vi "FlexMag - 23-03-2023.vi"() -> ()   [LabVIEW 2018] (continued)
                                stop <- w20767 stop-if-true
                                n15578 = Greater Or Equal?(x=w20771, y=200) -> (x >= y?=w20773:bool)
                                n15579 = case shown="True" w20773 {
                                frame False {
                                }
                                frame True {
                                n15580 = local write "ch2 pumpdown error"(TRUE ("ch1 pumpdown error")) -> ()
                                n15581 = local write "Warning Message"("CH2 PumpDown process  is canceled !\nCH2 PC GV couldn't be opened" ("Warning Message")) -> ()
                                }
                                }
                                n15582 = local read "ch2 pumpdown alg"() -> (w20770:bool)
                                n15583 = local read "ch2_pcgv_gui"() -> (w20766:bool)
                                n15584 = local read "abort ch2"() -> (w20768:bool)
                                n15585 = Wait Until Next ms Multiple(millisecond multiple=u32 200) -> ()  [unwired: 1 out]
                                n15586 = Not(x=w20770) -> (.not. x?=w20769:bool)
                                n15587 = Compound Arithmetic op=OR(w20766, w20768, w20769) -> (w20767:bool)
                                }
                                }
                                }
                              }
                              frame #4 {
                                n15588 = local read "ch2 pumpdown alg"() -> (w20776:bool)
                                n15589 = case shown="True" w20776 {
                                frame False {
                                }
                                frame True {
                                n15590 = local write "ch2 pc gv open led"(TRUE ("ch1 tp bv open led")) -> ()
                                n15591 = Wait (ms)(milliseconds to wait=u32 1000) -> ()  [unwired: 1 out]
                                }
                                }
                              }
                            }
                          }
                        }
                      }
                      frame True {
                      }
                    }
                  }
                }
              }
              frame #16 {
                n15592 = stacked-sequence {
                  frame #0 {
                    n15593 = local read "ch2 pumpdown alg"() -> (w20779:bool)
                    n15594 = case shown="True" w20779 {
                      frame False {
                      }
                      frame True {
                        n15595 = local read "abort ch2"() -> (w20780:bool)
                        n15596 = case shown="False" w20780 {
                          frame False {
                            n15597 = local write "CH2_PL_ATM_DO"(TRUE ("CH1_PL_ATM_DO")) -> ()
                            n15598 = Wait (ms)(milliseconds to wait=u32 2000) -> ()  [unwired: 1 out]
                          }
                          frame True {
                          }
                        }
                      }
                    }
                  }
                  frame #1 {
                    n15599 = local read "ch2 pumpdown alg"() -> (w20783:bool)
                    n15600 = case shown="True" w20783 {
                      frame False {
                      }
                      frame True {
                        n15601 = local read "abort ch2"() -> (w20784:bool)
                        n15602 = case shown="False" w20784 {
                          frame False {
                            n15603 = local write "CH2_CH_ATM_DO"(TRUE ("CH1_CH_ATM_DO")) -> ()
                            n15604 = Wait (ms)(milliseconds to wait=u32 2000) -> ()  [unwired: 1 out]
                          }
                          frame True {
                          }
                        }
                      }
                    }
                  }
                }
              }
              frame #17 {
                # "mp start"
                n15605 = local read "ch2 pumpdown alg"() -> (w20787:bool)
                n15606 = case shown="True" w20787 {
                  frame False {
                  }
                  frame True {
                    n15607 = local read "abort ch2"() -> (w20788:bool)
                    n15608 = case shown="False" w20788 {
                      frame False {
                        n15609 = while {
                          i -> [w20793]
                          stop <- w20797 stop-if-true
                          n15610 = Greater?(x=w20793, y=100) -> (0:w20789:bool)
                          n15611 = case shown="True" w20789 {
                            frame False {
                            }
                            frame True {
                              n15612 = local write "Warning Message"("CH2 PumpDown process  is canceled !\nCH2 MP couldn't be started" ("Warning Message")) -> ()
                              n15613 = local write "ch2 pumpdown error"(TRUE ("ch1 pumpdown error")) -> ()
                            }
                          }
                          n15614 = local read "CH2_MP_DI"() -> (w20791:bool)
                          n15615 = case shown="False" w20791 {
                            tunnel: [FALSE TRUE] -> w20790
                            frame False {
                              n15616 = Wait Until Next ms Multiple(millisecond multiple=u32 200) -> ()  [unwired: 1 out]
                              n15617 = local write "CH2_MP_DO"(TRUE ("CH1_MP_DO")) -> ()
                            }
                            frame True {
                            }
                          }
                          n15618 = local read "ch2 pumpdown alg"() -> (w20796:bool)
                          n15619 = local read "abort ch2"() -> (w20794:bool)
                          n15620 = Not(x=w20796) -> (.not. x?=w20795:bool)
                          n15621 = Compound Arithmetic op=OR(w20790, w20794, w20795) -> (w20797:bool)
                        }
                      }
                      frame True {
                      }
                    }
                  }
                }
              }
              frame #18 {
                n15622 = local read "ch2 pumpdown alg"() -> (w20804:bool)
                n15623 = case shown="True" w20804 {
                  frame False {
                  }
                  frame True {
                    n15624 = local read "abort ch2"() -> (w20805:bool)
                    n15625 = case shown="False" w20805 {
                      frame False {
                        n15626 = local write "ch2 mp start led"(TRUE ("ch1 ch vbv close")) -> ()
                        n15627 = Wait (ms)(milliseconds to wait=u32 1000) -> ()  [unwired: 1 out]
                      }
                      frame True {
                      }
                    }
                  }
                }
              }
              frame #19 {
                # "pl pg check"
                n15628 = local read "ch2 pumpdown alg"() -> (w20808:bool)
                n15629 = case shown="True" w20808 {
                  frame False {
                  }
                  frame True {
                    n15630 = local read "abort ch2"() -> (w20809:bool)
                    n15631 = case shown="False" w20809 {
                      frame False {
                        n15632 = while {
                          i -> [w20816]
                          stop <- w20820 stop-if-true
                          # "30 min"
                          n15633 = Greater?(x=w20816, y=9000) -> (0:w20813:bool)
                          n15634 = case shown="True" w20813 {
                            frame False {
                            }
                            frame True {
                              n15635 = local write "Warning Message"("CH2 PumpDown process  is canceled !\nCH2 PL Pressure couldn't be reached under 0.5 Torr" ("Warning Message")) -> ()
                              n15636 = local write "ch2 pumpdown error"(TRUE ("ch1 pumpdown error")) -> ()
                            }
                          }
                          n15637 = local read "ch2 pl pg  torr"() -> (w20812:dbl)
                          n15638 = Less?(x=w20812, y=0.7) -> (x < y?=w20810:bool)
                          n15639 = case shown="False" w20810 {
                            tunnel: [FALSE TRUE] -> w20814
                            frame False {
                              n15640 = Wait Until Next ms Multiple(millisecond multiple=u32 200) -> ()  [unwired: 1 out]
                            }
                            frame True {
                            }
                          }
                          n15641 = local read "ch2 pumpdown alg"() -> (w20819:bool)
                          n15642 = local read "abort ch2"() -> (w20817:bool)
                          n15643 = Not(x=w20819) -> (.not. x?=w20818:bool)
                          n15644 = Compound Arithmetic op=OR(w20814, w20817, w20818) -> (w20820:bool)
                        }
                      }
                      frame True {
                      }
                    }
                  }
                }
              }
              frame #20 {
                n15645 = local read "ch2 pumpdown alg"() -> (w20826:bool)
                n15646 = case shown="True" w20826 {
                  frame False {
                  }
                  frame True {
                    n15647 = local read "abort ch2"() -> (w20827:bool)
                    n15648 = case shown="False" w20827 {
                      frame False {
                        n15649 = local write "ch2 pl press under 0.05 T led"(TRUE ("ch1 ch vbv close")) -> ()
                        n15650 = Wait (ms)(milliseconds to wait=u32 1000) -> ()  [unwired: 1 out]
                      }
                      frame True {
                      }
                    }
                  }
                }
              }
              frame #21 {
                # "tp bv open"
                n15651 = local read "ch2 pumpdown alg"() -> (w20830:bool)
                n15652 = case shown="True" w20830 {
                  frame False {
                  }
                  frame True {
                    n15653 = local read "abort ch2"() -> (w20831:bool)
                    n15654 = case shown="False" w20831 {
                      frame False {
                        n15655 = while {
                          i -> [w20836]
                          stop <- w20840 stop-if-true
                          n15656 = Greater?(x=w20836, y=100) -> (0:w20832:bool)
                          n15657 = case shown="True" w20832 {
                            frame False {
                            }
                            frame True {
                              n15658 = local write "Warning Message"("CH2 PumpDown process  is canceled !\nCH2 TP BV couldn't be opened" ("Warning Message")) -> ()
                              n15659 = local write "ch2 pumpdown error"(TRUE ("ch1 pumpdown error")) -> ()
                            }
                          }
                          n15660 = local read "CH2_TP_BV_DI"() -> (w20834:bool)
                          n15661 = case shown="False" w20834 {
                            tunnel: [FALSE TRUE] -> w20833
                            frame False {
                              n15662 = Wait Until Next ms Multiple(millisecond multiple=u32 200) -> ()  [unwired: 1 out]
                              n15663 = local write "CH2_TP_BV_DO"(TRUE ("CH1_MP_DO")) -> ()
                            }
                            frame True {
                            }
                          }
                          n15664 = local read "ch2 pumpdown alg"() -> (w20839:bool)
                          n15665 = local read "abort ch2"() -> (w20837:bool)
                          n15666 = Not(x=w20839) -> (.not. x?=w20838:bool)
                          n15667 = Compound Arithmetic op=OR(w20833, w20837, w20838) -> (w20840:bool)
                        }
                      }
                      frame True {
                      }
                    }
                  }
                }
              }
              frame #22 {
                n15668 = local read "ch2 pumpdown alg"() -> (w20847:bool)
                n15669 = case shown="True" w20847 {
                  frame False {
                  }
                  frame True {
                    n15670 = local read "abort ch2"() -> (w20848:bool)
                    n15671 = case shown="False" w20848 {
                      frame False {
                        n15672 = local write "ch2 tp bv open led"(TRUE ("ch1 ch vbv close")) -> ()
                        n15673 = Wait (ms)(milliseconds to wait=u32 1000) -> ()  [unwired: 1 out]
                      }
                      frame True {
                      }
                    }
                  }
                }
              }
              frame #23 {
                # "pc gv open"
                n15674 = local read "ch2 pumpdown alg"() -> (w20851:bool)
                n15675 = case shown="True" w20851 {
                  frame False {
                  }
                  frame True {
                    n15676 = local read "abort ch2"() -> (w20852:bool)
                    n15677 = case shown="False" w20852 {
                      frame False {
                        n15678 = stacked-sequence {
                          frame #0 {
                            n15679 = local read "ch2 pumpdown alg"() -> (w20853:bool)
                            n15680 = case shown="True" w20853 {
                              frame False {
                              }
                              frame True {
                                n15681 = flat-sequence {
                                frame #0 {
                                n15682 = local write "pcgv2 auto open"(TRUE ("pcgv1 auto open")) -> ()
                                }
                                frame #1 {
                                n15683 = Wait (ms)(milliseconds to wait=u32 2000) -> ()  [unwired: 1 out]
                                }
                                frame #2 {
                                n15684 = local write "pcgv2 auto open"(TRUE ("pcgv1 auto open")) -> ()
                                }
                                }
                              }
                            }
                          }
                          frame #1 {
                            n15685 = while {
                              i -> [w20863]
                              stop <- w20859 stop-if-true
                              n15686 = Greater Or Equal?(x=w20863, y=200) -> (x >= y?=w20865:bool)
                              n15687 = case shown="True" w20865 {
                                frame False {
                                }
                                frame True {
                                n15688 = local write "ch2 pumpdown error"(TRUE ("ch1 pumpdown error")) -> ()
                                n15689 = local write "Warning Message"("CH2 PumpDown process  is canceled !\nCH2 PC GV couldn't be opened" ("Warning Message")) -> ()
                                }
                              }
                              n15690 = local read "ch2 pumpdown alg"() -> (w20862:bool)
                              n15691 = local read "ch2_pcgv_gui"() -> (w20858:bool)
                              n15692 = local read "abort ch2"() -> (w20860:bool)
                              n15693 = Wait Until Next ms Multiple(millisecond multiple=u32 200) -> ()  [unwired: 1 out]
                              n15694 = Not(x=w20862) -> (.not. x?=w20861:bool)
                              n15695 = Compound Arithmetic op=OR(w20858, w20860, w20861) -> (w20859:bool)
                            }
                          }
                        }
                      }
                      frame True {
                      }
                    }
                  }
                }
              }
              frame #24 {
                n15696 = local read "ch2 pumpdown alg"() -> (w20868:bool)
                n15697 = case shown="True" w20868 {
                  frame False {
                  }
                  frame True {
                    n15698 = local read "abort ch2"() -> (w20869:bool)
                    n15699 = case shown="False" w20869 {
                      frame False {
                        n15700 = local write "ch2 pc gv open led"(TRUE ("ch1 ch vbv close")) -> ()
                        n15701 = Wait (ms)(milliseconds to wait=u32 1000) -> ()  [unwired: 1 out]
                      }
                      frame True {
                      }
                    }
                  }
                }
              }
              frame #25 {
                # "ch pressure check"
                n15702 = local read "ch2 pumpdown alg"() -> (w20872:bool)
                n15703 = case shown="True" w20872 {
                  frame False {
                  }
                  frame True {
                    n15704 = local read "abort ch2"() -> (w20873:bool)
                    n15705 = case shown="False" w20873 {
                      frame False {
                        n15706 = while {
                          i -> [w20880]
                          stop <- w20884 stop-if-true
                          # "30 min"
                          n15707 = Greater?(x=w20880, y=9000) -> (0:w20877:bool)
                          n15708 = case shown="True" w20877 {
                            frame False {
                            }
                            frame True {
                              n15709 = local write "Warning Message"("CH2 PumpDown process  is canceled !\nCH2 CH Pressure couldn't be reached under 0.5 Torr" ("Warning Message")) -> ()
                              n15710 = local write "ch2 pumpdown error"(TRUE ("ch1 pumpdown error")) -> ()
                            }
                          }
                          n15711 = local read "ch2 ch pg torr"() -> (w20876:dbl)
                          n15712 = Less Or Equal?(x=w20876, y=0.5) -> (x <= y?=w20874:bool)
                          n15713 = case shown="False" w20874 {
                            tunnel: [FALSE TRUE] -> w20878
                            frame False {
                              n15714 = Wait Until Next ms Multiple(millisecond multiple=u32 200) -> ()  [unwired: 1 out]
                            }
                            frame True {
                            }
                          }
                          n15715 = local read "ch2 pumpdown alg"() -> (w20883:bool)
                          n15716 = local read "abort ch2"() -> (w20881:bool)
                          n15717 = Not(x=w20883) -> (.not. x?=w20882:bool)
                          n15718 = Compound Arithmetic op=OR(w20878, w20881, w20882) -> (w20884:bool)
                        }
                      }
                      frame True {
                      }
                    }
                  }
                }
              }
              frame #26 {
                n15719 = local read "ch2 pumpdown alg"() -> (w20890:bool)
                n15720 = case shown="True" w20890 {
                  frame False {
                  }
                  frame True {
                    n15721 = local read "abort ch2"() -> (w20891:bool)
                    n15722 = case shown="False" w20891 {
                      frame False {
                        n15723 = local write "ch2 ch press under 0.5 T led"(TRUE ("ch1 ch pressure led")) -> ()
                        n15724 = Wait (ms)(milliseconds to wait=u32 1000) -> ()  [unwired: 1 out]
                      }
                      frame True {
                      }
                    }
                  }
                }
              }
              frame #27 {
                # "ch 1 pressure check\nfor trns bp bv"
                n15725 = local read "ch2 pumpdown alg"() -> (w20894:bool)
                n15726 = case shown="True" w20894 {
                  frame False {
                  }
                  frame True {
                    n15727 = local read "abort ch2"() -> (w20895:bool)
                    n15728 = case shown="False" w20895 {
                      frame False {
                        n15729 = local read "ch1 ch pg torr"() -> (w20898:dbl)
                        n15730 = Less Or Equal?(x=w20898, y=0.5) -> (x <= y?=w20896:bool)
                        n15731 = case shown="True" w20896 {
                          frame False {
                          }
                          frame True {
                            n15732 = stacked-sequence {
                              frame #0 {
                                n15733 = while {
                                i -> [w20903]
                                stop <- w20907 stop-if-true
                                n15734 = Greater?(x=w20903, y=100) -> (0:w20900:bool)
                                n15735 = case shown="True" w20900 {
                                frame False {
                                }
                                frame True {
                                n15736 = local write "ch2 pumpdown error"(TRUE ("ch1 pumpdown error")) -> ()
                                n15737 = local write "Warning Message"("CH2 PumpDown process  is canceled !\nCH2 Trns BP Right couldn't be opened" ("Warning Message")) -> ()
                                }
                                }
                                n15738 = local read "CH2_Trns_BP_Right_DI"() -> (w20899:bool)
                                n15739 = case shown="False" w20899 {
                                tunnel: [FALSE TRUE] -> w20901
                                frame False {
                                n15740 = local write "CH2_Trns_BP_Right_DO"(TRUE ("CH1_Trns_BP_Left_DO")) -> ()
                                n15741 = Wait Until Next ms Multiple(millisecond multiple=u32 200) -> ()  [unwired: 1 out]
                                }
                                frame True {
                                }
                                }
                                n15742 = local read "ch2 pumpdown alg"() -> (w20906:bool)
                                n15743 = local read "abort ch2"() -> (w20904:bool)
                                n15744 = Not(x=w20906) -> (.not. x?=w20905:bool)
                                n15745 = Compound Arithmetic op=OR(w20901, w20904, w20905) -> (w20907:bool)
                                }
                              }
                              frame #1 {
                                n15746 = local read "ch2 pumpdown alg"() -> (w20914:bool)
                                n15747 = case shown="True" w20914 {
                                frame False {
                                }
                                frame True {
                                n15748 = local read "abort ch2"() -> (w20915:bool)
                                n15749 = case shown="False" w20915 {
                                frame False {
                                n15750 = local write "ch2 trns bp right open led"(TRUE ("ch1 tp start led")) -> ()
                                n15751 = local write "ch1_2 vacuum level"("VACUUM" ("ch3_4 vacuum level")) -> ()
                                n15752 = Wait (ms)(milliseconds to wait=u32 1000) -> ()  [unwired: 1 out]
                                }
                                frame True {
                                }
                                }
                                }
                                }
                              }
                              frame #2 {
                                n15753 = while {
                                i -> [w20921]
                                stop <- w20923 stop-if-true
                                n15754 = local read "ch2 pumpdown alg"() -> (w20924:bool)
                                n15755 = Wait Until Next ms Multiple(millisecond multiple=u32 200) -> ()  [unwired: 1 out]
                                n15756 = local read "abort ch2"() -> (w20926:bool)
                                n15757 = Greater?(x=w20921, y=100) -> (0:w20920:bool)
                                n15758 = Not(x=w20924) -> (.not. x?=w20925:bool)
                                n15759 = Compound Arithmetic op=OR(w20920, w20926, w20925) -> (w20923:bool)
                                }
                              }
                            }
                          }
                        }
                      }
                      frame True {
                      }
                    }
                  }
                }
              }
              frame #28 {
              }
              frame #29 {
                # "ch 3 pressure check\nfor trns bp bv"
                n15760 = local read "ch2 pumpdown alg"() -> (w20927:bool)
                n15761 = case shown="True" w20927 {
                  frame False {
                  }
                  frame True {
                    n15762 = local read "abort ch2"() -> (w20928:bool)
                    n15763 = case shown="False" w20928 {
                      frame False {
                        n15764 = local read "ch3 ch pg torr"() -> (w20931:dbl)
                        n15765 = Less Or Equal?(x=w20931, y=0.5) -> (x <= y?=w20929:bool)
                        n15766 = case shown="True" w20929 {
                          frame False {
                          }
                          frame True {
                            n15767 = stacked-sequence {
                              frame #0 {
                                n15768 = while {
                                i -> [w20936]
                                stop <- w20940 stop-if-true
                                n15769 = Greater?(x=w20936, y=100) -> (0:w20933:bool)
                                n15770 = case shown="True" w20933 {
                                frame False {
                                }
                                frame True {
                                n15771 = local write "Warning Message"("CH2 PumpDown process  is canceled !\nCH2 Trns BP Left couldn't be opened" ("Warning Message")) -> ()
                                n15772 = local write "ch2 pumpdown error"(TRUE ("ch1 pumpdown error")) -> ()
                                }
                                }
                                n15773 = local read "CH2_Trns_BP_Left_DI"() -> (w20932:bool)
                                n15774 = case shown="False" w20932 {
                                tunnel: [FALSE TRUE] -> w20934
                                frame False {
                                n15775 = local write "CH2_Trns_BP_Left_DO"(TRUE ("CH1_Trns_BP_Left_DO")) -> ()
                                n15776 = Wait Until Next ms Multiple(millisecond multiple=u32 200) -> ()  [unwired: 1 out]
                                }
                                frame True {
                                }
                                }
                                n15777 = local read "ch2 pumpdown alg"() -> (w20939:bool)
                                n15778 = local read "abort ch2"() -> (w20937:bool)
                                n15779 = Not(x=w20939) -> (.not. x?=w20938:bool)
                                n15780 = Compound Arithmetic op=OR(w20934, w20937, w20938) -> (w20940:bool)
                                }
                              }
                              frame #1 {
                                n15781 = local read "ch2 pumpdown alg"() -> (w20947:bool)
                                n15782 = case shown="True" w20947 {
                                frame False {
                                }
                                frame True {
                                n15783 = local read "abort ch2"() -> (w20948:bool)
                                n15784 = case shown="False" w20948 {
                                frame False {
                                n15785 = local write "ch2 trns bp left open led"(TRUE ("ch1 tp start led")) -> ()
                                n15786 = local write "ch2_3 vacuum level"("VACUUM" ("ch3_4 vacuum level")) -> ()
                                n15787 = Wait (ms)(milliseconds to wait=u32 1000) -> ()  [unwired: 1 out]
                                }
                                frame True {
                                }
                                }
                                }
                                }
                              }
                              frame #2 {
                                n15788 = while {
                                i -> [w20954]
                                stop <- w20956 stop-if-true
                                n15789 = Wait Until Next ms Multiple(millisecond multiple=u32 200) -> ()  [unwired: 1 out]
                                n15790 = local read "ch1 pumpdown alg"() -> (w20957:bool)
                                n15791 = local read "abort ch1"() -> (w20959:bool)
                                n15792 = Greater?(x=w20954, y=100) -> (0:w20953:bool)
                                n15793 = Not(x=w20957) -> (.not. x?=w20958:bool)
                                n15794 = Compound Arithmetic op=OR(w20953, w20959, w20958) -> (w20956:bool)
                                }
                              }
                            }
                          }
                        }
                      }
                      frame True {
                      }
                    }
                  }
                }
              }
              frame #30 {
                # "ch pressure check"
                n15795 = local read "ch2 pumpdown alg"() -> (w20960:bool)
                n15796 = case shown="True" w20960 {
                  frame False {
                  }
                  frame True {
                    n15797 = local read "abort ch2"() -> (w20961:bool)
                    n15798 = case shown="False" w20961 {
                      frame False {
                        n15799 = while {
                          i -> [w20968]
                          stop <- w20972 stop-if-true
                          # "20 min"
                          n15800 = Greater?(x=w20968, y=6000) -> (0:w20965:bool)
                          n15801 = case shown="True" w20965 {
                            frame False {
                            }
                            frame True {
                              n15802 = local write "Warning Message"("CH2 PumpDown process  is canceled !\nCH2 CH Pressure couldn't be reached under 0.2 Torr" ("Warning Message")) -> ()
                              n15803 = local write "ch2 pumpdown error"(TRUE ("ch1 pumpdown error")) -> ()
                            }
                          }
                          n15804 = local read "ch2 ch pg torr"() -> (w20964:dbl)
                          n15805 = Less Or Equal?(x=w20964, y=0.5) -> (x <= y?=w20962:bool)
                          n15806 = case shown="True" w20962 {
                            tunnel: [FALSE TRUE] -> w20966
                            frame False {
                              n15807 = Wait Until Next ms Multiple(millisecond multiple=u32 200) -> ()  [unwired: 1 out]
                            }
                            frame True {
                            }
                          }
                          n15808 = local read "ch2 pumpdown alg"() -> (w20971:bool)
                          n15809 = local read "abort ch2"() -> (w20969:bool)
                          n15810 = Not(x=w20971) -> (.not. x?=w20970:bool)
                          n15811 = Compound Arithmetic op=OR(w20966, w20969, w20970) -> (w20972:bool)
                        }
                      }
                      frame True {
                      }
                    }
                  }
                }
              }
              frame #31 {
                # "tp start"
                n15812 = local read "ch2 pumpdown alg"() -> (w20978:bool)
                n15813 = case shown="True" w20978 {
                  frame False {
                  }
                  frame True {
                    n15814 = local read "abort ch2"() -> (w20979:bool)
                    n15815 = case shown="False" w20979 {
                      frame False {
                        n15816 = stacked-sequence {
                          frame #0 {
                            n15817 = flat-sequence {
                              frame #0 {
                                n15818 = local write "Tp2 auto start"(TRUE ("Tp1 auto start")) -> ()
                                n15819 = Wait (ms)(milliseconds to wait=u32 100) -> ()  [unwired: 1 out]
                              }
                              frame #1 {
                                n15820 = Wait (ms)(milliseconds to wait=u32 2000) -> ()  [unwired: 1 out]
                              }
                              frame #2 {
                                n15821 = disable-structure shown="Disabled" {
                                frame Disabled {
                                n15822 = local write "Tp1 Start initial"(TRUE ("Tp1 Start initial")) -> ()
                                }
                                frame Enabled {
                                }
                                }
                              }
                              frame #3 {
                                n15823 = Wait (ms)(milliseconds to wait=u32 2000) -> ()  [unwired: 1 out]
                              }
                              frame #4 {
                                n15824 = local write "Tp2 auto low speed"(TRUE ("Tp1 auto start")) -> ()
                                n15825 = Wait (ms)(milliseconds to wait=u32 100) -> ()  [unwired: 1 out]
                              }
                            }
                          }
                          frame #1 {
                            n15826 = while {
                              i -> [w20995]
                              stop <- w20989 stop-if-true
                              # "200 sec ?"
                              n15827 = Greater Or Equal?(x=w20995, y=1000) -> (x >= y?=w20988:bool)
                              n15828 = case shown="True" w20988 {
                                frame False {
                                }
                                frame True {
                                n15829 = local write "Warning Message"("CH2 PumpDown process  is canceled !\nCH2 TP couldn't be started" ("Warning Message")) -> ()
                                n15830 = local write "ch2 pumpdown error"(TRUE ("ch1 pumpdown error")) -> ()
                                }
                              }
                              n15831 = local read "ch2 pumpdown alg"() -> (w20992:bool)
                              n15832 = local read "ch2_tp_gui"() -> (w20987:bool)
                              n15833 = local read "abort ch2"() -> (w20990:bool)
                              n15834 = Not(x=w20992) -> (.not. x?=w20991:bool)
                              n15835 = Wait Until Next ms Multiple(millisecond multiple=u32 200) -> ()  [unwired: 1 out]
                              n15836 = Compound Arithmetic op=OR(w20987, w20990, w20991) -> (w20989:bool)
                            }
                          }
                        }
                      }
                      frame True {
                      }
                    }
                  }
                }
              }
              frame #32 {
                n15837 = local read "ch2 pumpdown alg"() -> (w20998:bool)
                n15838 = case shown="True" w20998 {
                  frame False {
                  }
                  frame True {
                    n15839 = local read "abort ch2"() -> (w20999:bool)
                    n15840 = case shown="False" w20999 {
                      frame False {
                        n15841 = local write "ch2 tp start led"(TRUE ("ch1 tp start led")) -> ()
                        n15842 = Wait (ms)(milliseconds to wait=u32 1000) -> ()  [unwired: 1 out]
                      }
                      frame True {
                      }
                    }
                  }
                }
              }
              frame #33 {
                n15843 = local read "ch2 pumpdown alg"() -> (w21002:bool)
                n15844 = case shown="True" w21002 {
                  frame False {
                  }
                  frame True {
                    n15845 = local read "abort ch2"() -> (w21003:bool)
                    n15846 = case shown="False" w21003 {
                      frame False {
                        n15847 = while {
                          i -> [w21010]
                          stop <- w21014 stop-if-true
                          # "30 min"
                          n15848 = Greater?(x=w21010, y=9000) -> (0:w21007:bool)
                          n15849 = case shown="True" w21007 {
                            frame False {
                            }
                            frame True {
                              n15850 = local write "Warning Message"("CH2 PumpDown process  is canceled !\nCH2 CH Pressure couldn't be reached under 0.01 Torr" ("Warning Message")) -> ()
                              n15851 = local write "ch2 pumpdown error"(TRUE ("ch1 pumpdown error")) -> ()
                            }
                          }
                          n15852 = local read "ch2 ch pg torr"() -> (w21006:dbl)
                          n15853 = Less Or Equal?(x=w21006, y=0.09) -> (x <= y?=w21004:bool)
                          n15854 = case shown="False" w21004 {
                            tunnel: [FALSE TRUE] -> w21008
                            frame False {
                              n15855 = Wait Until Next ms Multiple(millisecond multiple=u32 200) -> ()  [unwired: 1 out]
                            }
                            frame True {
                            }
                          }
                          n15856 = local read "ch2 pumpdown alg"() -> (w21013:bool)
                          n15857 = local read "abort ch2"() -> (w21011:bool)
                          n15858 = Not(x=w21013) -> (.not. x?=w21012:bool)
                          n15859 = Compound Arithmetic op=OR(w21008, w21011, w21012) -> (w21014:bool)
                        }
                      }
                      frame True {
                      }
                    }
                  }
                }
              }
              frame #34 {
                n15860 = local read "ch2 pumpdown alg"() -> (w21020:bool)
                n15861 = case shown="True" w21020 {
                  frame False {
                  }
                  frame True {
                    n15862 = local read "abort ch2"() -> (w21021:bool)
                    n15863 = case shown="False" w21021 {
                      frame False {
                        n15864 = local write "ch2 ch press under 0.01 T led"(TRUE ("ch1 pressure under 0.05 torr led")) -> ()
                        n15865 = Wait (ms)(milliseconds to wait=u32 1000) -> ()  [unwired: 1 out]
                      }
                      frame True {
                      }
                    }
                  }
                }
              }
              frame #35 {
                n15866 = local read "ch2 pumpdown alg"() -> (w21024:bool)
                n15867 = case shown="True" w21024 {
                  frame False {
                  }
                  frame True {
                    n15868 = local read "abort ch2"() -> (w21025:bool)
                    n15869 = case shown="False" w21025 {
                      frame False {
                        n15870 = stacked-sequence {
                          frame #0 {
                            n15871 = while {
                              i -> [w21030]
                              stop <- w21034 stop-if-true
                              n15872 = Greater?(x=w21030, y=200) -> (0:w21027:bool)
                              n15873 = case shown="True" w21027 {
                                frame False {
                                }
                                frame True {
                                n15874 = local write "Warning Message"("CH2 PumpDown process  is canceled !\nCH2 CC couldn't be opened" ("Warning Message")) -> ()
                                n15875 = local write "ch2 pumpdown error"(TRUE ("ch1 pumpdown error")) -> ()
                                }
                              }
                              n15876 = local read "CH2_CC_DI"() -> (w21026:bool)
                              n15877 = case shown="False" w21026 {
                                tunnel: [FALSE TRUE] -> w21028
                                frame False {
                                n15878 = Wait Until Next ms Multiple(millisecond multiple=u32 200) -> ()  [unwired: 1 out]
                                n15879 = local write "CH2_CC_DO"(TRUE ("CH1_CC_DO")) -> ()
                                }
                                frame True {
                                }
                              }
                              n15880 = local read "ch2 pumpdown alg"() -> (w21033:bool)
                              n15881 = local read "abort ch2"() -> (w21031:bool)
                              n15882 = Not(x=w21033) -> (.not. x?=w21032:bool)
                              n15883 = Compound Arithmetic op=OR(w21028, w21031, w21032) -> (w21034:bool)
                            }
                          }
                          frame #1 {
                            n15884 = while {
                              i -> [w21043]
                              stop <- w21045 stop-if-true
                              n15885 = local read "ch2 pumpdown alg"() -> (w21046:bool)
                              n15886 = local read "abort ch2"() -> (w21048:bool)
                              n15887 = Greater Or Equal?(x=w21043, y=300) -> (x >= y?=w21041:bool)
                              n15888 = Not(x=w21046) -> (.not. x?=w21047:bool)
                              n15889 = Compound Arithmetic op=OR(w21041, w21048, w21047) -> (w21045:bool)
                              n15890 = Wait Until Next ms Multiple(millisecond multiple=u32 200) -> ()  [unwired: 1 out]
                            }
                          }
                        }
                      }
                      frame True {
                      }
                    }
                  }
                }
              }
              frame #36 {
                n15891 = local read "ch2 pumpdown alg"() -> (w21049:bool)
                n15892 = case shown="True" w21049 {
                  frame False {
                  }
                  frame True {
                    n15893 = local read "abort ch2"() -> (w21050:bool)
                    n15894 = case shown="False" w21050 {
                      frame False {
                        n15895 = local write "ch2 cc open led"(TRUE ("ch1 ch cc open led")) -> ()
                        n15896 = Wait (ms)(milliseconds to wait=u32 1000) -> ()  [unwired: 1 out]
                      }
                      frame True {
                      }
                    }
                  }
                }
              }
              frame #37 {
                n15897 = local read "ch2 pumpdown alg"() -> (w21053:bool)
                n15898 = case shown="True" w21053 {
                  frame False {
                  }
                  frame True {
                    n15899 = local read "abort ch2"() -> (w21054:bool)
                    n15900 = case shown="False" w21054 {
                      frame False {
                        n15901 = while {
                          i -> [w21065]
                          stop <- w21069 stop-if-true
                          # "60 min"
                          n15902 = Multiply(x=27000 ("y"), y=3) -> (x*y=w21055:i32)
                          n15903 = Greater?(x=w21065, y=w21055) -> (0:w21063:bool)
                          n15904 = case shown="True" w21063 {
                            frame False {
                            }
                            frame True {
                              n15905 = local write "Warning Message"("CH2 PumpDown process  is canceled !\nCH2 CH Pressure couldn't be reached to desired pressure" ("Warning Message")) -> ()
                              n15906 = local write "ch2 pumpdown error"(TRUE ("ch1 pumpdown error")) -> ()
                            }
                          }
                          n15907 = local read "ch2 cc torr"() -> (w21062:dbl)
                          n15908 = Multiply(x=0.75, y="ch2 desired pressure") -> (x*y=w21059:dbl)
                          n15909 = Less Or Equal?(x=w21062, y=w21059) -> (x <= y?=w21061:bool)
                          n15910 = case shown="False" w21061 {
                            tunnel: [FALSE TRUE] -> w21064
                            frame False {
                              n15911 = Wait Until Next ms Multiple(millisecond multiple=u32 200) -> ()  [unwired: 1 out]
                            }
                            frame True {
                            }
                          }
                          n15912 = local read "ch2 pumpdown alg"() -> (w21068:bool)
                          n15913 = local read "abort ch2"() -> (w21066:bool)
                          n15914 = Not(x=w21068) -> (.not. x?=w21067:bool)
                          n15915 = Compound Arithmetic op=OR(w21064, w21066, w21067) -> (w21069:bool)
                        }
                      }
                      frame True {
                      }
                    }
                  }
                }
              }
              frame #38 {
                n15916 = local read "ch2 pumpdown alg"() -> (w21075:bool)
                n15917 = case shown="True" w21075 {
                  frame False {
                  }
                  frame True {
                    n15918 = local read "abort ch2"() -> (w21076:bool)
                    n15919 = case shown="False" w21076 {
                      frame False {
                        n15920 = local write "ch2 desired pressure led"(TRUE ("ch1 pumdown completed led")) -> ()
                        n15921 = Wait (ms)(milliseconds to wait=u32 1000) -> ()  [unwired: 1 out]
                      }
                      frame True {
                      }
                    }
                  }
                }
              }
              frame #39 {
                n15922 = local read "ch2 pumpdown alg"() -> (w21079:bool)
                n15923 = case shown="True" w21079 {
                  frame False {
                  }
                  frame True {
                    n15924 = local read "abort ch2"() -> (w21080:bool)
                    n15925 = case shown="False" w21080 {
                      frame False {
                        w21082 = TRUE ("Buzzer DO")
                        n15926 = local write "Buzzer DO"(w21082) -> ()
                        n15927 = local write "ch2 pd completed led"(w21082) -> ()
                        n15928 = local write "CH2_BG_BV_DO"(TRUE ("CH1_BG_BV_DO")) -> ()
                        n15929 = Wait (ms)(milliseconds to wait=u32 3000) -> ()  [unwired: 1 out]
                        n15930 = local write "System Status"("CH2 PUMPDOWN PROCESS COMPLETED" ("System Status")) -> ()
                      }
                      frame True {
                      }
                    }
                  }
                }
              }
              frame #40 {
                n15931 = local read "ch2 pumpdown alg"() -> (w21085:bool)
                n15932 = case shown="True" w21085 {
                  frame False {
                  }
                  frame True {
                    n15933 = local read "abort ch2"() -> (w21086:bool)
                    n15934 = case shown="False" w21086 {
                      frame False {
                        w21088 = FALSE ("Buzzer DO")
                        n15935 = local write "Buzzer DO"(w21088) -> ()
                        n15936 = local write "ch2 pumpdown alg"(w21088) -> ()
                        n15937 = local write "Pump Down CH2"(w21088) -> ()
                        n15938 = Wait (ms)(milliseconds to wait=u32 3000) -> ()  [unwired: 1 out]
                        n15939 = local write "System Status"("SEMI-AUTOMATIC MODE " ("System Status")) -> ()
                      }
                      frame True {
                      }
                    }
                  }
                }
              }
            }
          }
          frame True {
          }
        }
      }
    }
    n15940 = case shown="True" "ch2 shutdown alg" {
      frame False {
      }
      frame True {
        n15941 = local read "abort ch2"() -> (w20169:bool)
        n15942 = case shown="False" w20169 {
          frame False {
            n15943 = stacked-sequence {
              frame #0 {
                n15944 = stacked-sequence {
                  frame #0 {
                    n15945 = local write "ch2 vent?"(FALSE ("ch1 vent?")) -> ()
                    n15946 = Wait (ms)(milliseconds to wait=u32 1000) -> ()  [unwired: 1 out]
                  }
                  frame #1 {
                    n15947 = local write "System Status"("CH2 SHUTDOWN PROCESS IN PROGRESS" ("System Status")) -> ()
                  }
                  frame #2 {
                    n15948 = Two Button Dialog(message="Do you want to Vent CH2 ?", 1:"No, SHUTDOWN only" ("F button name (\"Cancel\")"), 2:"Yes, VENT! CH2" ("T button name (\"OK\")")) -> (T button?=w20173:bool)
                    "ch2 vent?" <- w20173
                    n15949 = case shown="True" w20173 {
                      frame False {
                      }
                      frame True {
                        w20177 = FALSE ("CH2_Trns_BP_Right_DO")
                        n15950 = local write "CH3_Trns_BP_Right_DO"(w20177) -> ()
                        n15951 = local write "CH1_Trns_BP_Left_DO"(w20177) -> ()
                      }
                    }
                  }
                }
              }
              frame #1 {
                # "ATMs close"
                n15952 = local read "ch2 shutdown alg"() -> (w20178:bool)
                n15953 = case shown="True" w20178 {
                  frame False {
                  }
                  frame True {
                    n15954 = local read "abort ch2"() -> (w20179:bool)
                    n15955 = case shown="False" w20179 {
                      frame False {
                        w20180 = FALSE ("CH1_PL_ATM_DO")
                        n15956 = local write "CH2_PL_ATM_DO"(w20180) -> ()
                        n15957 = local write "CH2_CH_ATM_DO"(w20180) -> ()
                        n15958 = Wait (ms)(milliseconds to wait=u32 3000) -> ()  [unwired: 1 out]
                      }
                      frame True {
                      }
                    }
                  }
                }
              }
              frame #2 {
                n15959 = local read "ch1 shutdown alg"() -> (w20182:bool)
                n15960 = case shown="True" w20182 {
                  frame False {
                  }
                  frame True {
                    n15961 = local read "abort ch1"() -> (w20183:bool)
                    n15962 = case shown="False" w20183 {
                      frame False {
                        n15963 = local write "ch2 sd atms close led"(TRUE ("ch1 sd cc close led")) -> ()
                        n15964 = Wait (ms)(milliseconds to wait=u32 1000) -> ()  [unwired: 1 out]
                      }
                      frame True {
                      }
                    }
                  }
                }
              }
              frame #3 {
                # "CC close"
                n15965 = local read "ch2 shutdown alg"() -> (w20186:bool)
                n15966 = case shown="True" w20186 {
                  frame False {
                  }
                  frame True {
                    n15967 = local read "abort ch2"() -> (w20187:bool)
                    n15968 = case shown="False" w20187 {
                      frame False {
                        n15969 = while {
                          i -> [w20192]
                          stop <- w20196 stop-if-true
                          n15970 = Greater?(x=w20192, y=100) -> (0:w20189:bool)
                          n15971 = case shown="True" w20189 {
                            frame False {
                            }
                            frame True {
                              n15972 = local write "Warning Message"("CH2 ShutDown process  is canceled !\nCH2 CC couldn't be closed" ("Warning Message")) -> ()
                              n15973 = local write "ch2 shutdown error"(TRUE ("ch1 pumpdown error")) -> ()
                            }
                          }
                          n15974 = local read "CH2_CC_DI"() -> (w20188:bool)
                          n15975 = case shown="True" w20188 {
                            tunnel: [TRUE FALSE] -> w20190
                            frame False {
                            }
                            frame True {
                              n15976 = Wait Until Next ms Multiple(millisecond multiple=u32 200) -> ()  [unwired: 1 out]
                              n15977 = local write "CH2_CC_DO"(FALSE ("CH1_CC_DO")) -> ()
                            }
                          }
                          n15978 = local read "ch2 shutdown alg"() -> (w20195:bool)
                          n15979 = local read "abort ch2"() -> (w20193:bool)
                          n15980 = Not(x=w20195) -> (.not. x?=w20194:bool)
                          n15981 = Compound Arithmetic op=OR(w20190, w20193, w20194) -> (w20196:bool)
                        }
                      }
                      frame True {
                      }
                    }
                  }
                }
              }
              frame #4 {
                n15982 = local read "ch2 shutdown alg"() -> (w20203:bool)
                n15983 = case shown="True" w20203 {
                  frame False {
                  }
                  frame True {
                    n15984 = local read "abort ch2"() -> (w20204:bool)
                    n15985 = case shown="False" w20204 {
                      frame False {
                        n15986 = local write "ch2 sd cc close led"(TRUE ("ch1 sd cc close led")) -> ()
                        n15987 = Wait (ms)(milliseconds to wait=u32 1000) -> ()  [unwired: 1 out]
                      }
                      frame True {
                      }
                    }
                  }
                }
              }
              frame #5 {
                # "bg bv close"
                n15988 = local read "ch2 shutdown alg"() -> (w20207:bool)
                n15989 = case shown="True" w20207 {
                  frame False {
                  }
                  frame True {
                    n15990 = local read "abort ch2"() -> (w20208:bool)
                    n15991 = case shown="False" w20208 {
                      frame False {
                        n15992 = while {
                          i -> [w20213]
                          stop <- w20217 stop-if-true
                          n15993 = Greater?(x=w20213, y=100) -> (0:w20210:bool)
                          n15994 = case shown="True" w20210 {
                            frame False {
                            }
                            frame True {
                              n15995 = local write "Warning Message"("CH2 ShutDown process  is canceled !\nCH2 BG BV couldn't be closed" ("Warning Message")) -> ()
                              n15996 = local write "ch2 shutdown error"(TRUE ("ch1 pumpdown error")) -> ()
                            }
                          }
                          n15997 = local read "CH2_BG_BV_DI"() -> (w20209:bool)
                          n15998 = case shown="True" w20209 {
                            tunnel: [TRUE FALSE] -> w20211
                            frame False {
                            }
                            frame True {
                              n15999 = Wait Until Next ms Multiple(millisecond multiple=u32 200) -> ()  [unwired: 1 out]
                              n16000 = local write "CH2_BG_BV_DO"(FALSE ("CH1_CC_DO")) -> ()
                            }
                          }
                          n16001 = local read "ch2 shutdown alg"() -> (w20216:bool)